vi "Modelo planta H2_V2.vi"() -> ()   [LabVIEW 2024]
uses:
  <vilib>/Modbus/master/Create Master Instance (TCP).vi
  <vilib>/Modbus/master/Modbus Master.lvclass
  <vilib>/OPCUA/NI OPC UA Client.lvlib
  SALICRU_MODBUS.lvlib
  S7-1200_OPCUA.lvlib
panel:
  out "x-y 2":u32
  out "error out 2":errorcluster
  out "error out":errorcluster
  in  "stop":bool
  out "x-y":u32
  in  "Tab Control":enum32{"Vista General", "Producción", "Energía"}(tab)
  out "EV5":bool caption="Not initialized"
  out "EV6":bool caption="Not initialized"
  out "EV4":bool caption="Not initialized"
  out "EV2":bool caption="Not initialized"
  out "EV3":bool caption="Idle"
  out "EV1":bool caption="Stand By"
  out "E2.2":bool caption="Not initialized"
  out "E2.3":bool caption="Not initialized"
  out "E2.14 2":bool caption="Not initialized"
  out "E1.2":bool caption="Not initialized"
  out "E1.3":bool caption="Idle"
  out "E1.1":bool caption="Stand By"
  out "Prod electrolizadores (display) 2":dbl format="%#.4g"
  out "Potenica Solar (Display) 2":dbl format="%#.2f"
  out "masa total G g 2":dbl format="%#.0f"
  out "P alta 2":dbl format="%.2f"
  out "P baja 2":dbl format="%.2f"
  out "masa total P g  2":dbl format="%#.1f"
  in  "SAI":bool caption="Line"
  out "Potenica Solar (Display) 3":dbl format="%#.2f"
  out "E2.1":bool caption="Not initialized"
  out "E2.2":bool caption="Not initialized"
  out "E1.2 2":bool caption="Idle"
  out "E1.1,2":bool caption="Stand By"
  out "E2.1 3":bool caption="Not initialized"
  out "E1.2":bool caption="Not initialized"
  out "Producció d'hidrogen":dbl(graph)
  out "Energia solar no utilitzada":dbl(graph)
  out "Pressió tanc baixa":dbl(graph)
  out "Potenica Solar (Display)":dbl format="%#.2f"
  out "Producción FC":dbl format="%#_2g"
  out "Prod electrolizadores (display)":dbl format="%#.4g"
  out "P baja":dbl format="%.2f"
  out "masa total G g":dbl format="%#.0f"
  out "Potència inversor solar":dbl(graph)
  out "Watimetro ARPA":dbl format="%#.1f"
  out "masa total P g":dbl format="%#.1f"
  out "Compresor":bool
  out "P alta":dbl format="%.2f"
  out "Tèrmic\nExtractors":bool
  out "Relé Seguretat":bool
  out "Sobretensions":bool
  out "Baliza verde":bool
  out "Baliza amarilla":bool
  out "Baliza roja":bool
  out "H2 generado Total":dbl format="%#.1f"
  out "Producción Solar toral":dbl format="%#.1f"
  out "Energía acum H2 verde":dbl format="%#.1f"
  out "H2 consumido en el lab":dbl=182.6 format="%#.1f"
  out "Energía solar diaría":dbl format="%#.1f"
  out "H2 generado dia":dbl format="%#.1f"
  out "Tank":dbl(slide) scale=0.0..10.0
  out "P tanq alta (barg)":dbl(graph)
  in  "Energía acum H2 verde inicio":dbl=527.0
  in  "Producción Solar total inicio":dbl=3421.0
  in  "H2 generado inicio":dbl=202.8
  out "g H2 consumidos por la FC":dbl
  out "g comprimidos":dbl
  in  "Caudal compresor":dbl
  out "P tanq baja (barg)":dbl(graph)
  in  "Presión ini Tanq baba":dbl=28.0
  in  "Presión ini Tanq alta":dbl=220.0
  out "Energía Solar no usada (kWh)":dbl(graph)
  out "H2 acumulado diario (g)":dbl(graph)
  out "Producción instalan (g/s)":dbl(graph)
  out "Electroli ON":dbl(graph)
  out "Potencia Consumo electroli instan. (kW)":dbl(graph)
  out "Producción diaria (g)":dbl
  out "Producción instalan (g/s)":dbl
  out "Electroli ON":dbl
  out "Potencia Solar Instanta (kW)":dbl(graph)
  # "g"
  # "bar"
  # "bar"
  # "kg"
  # "kWh"
  # "kWh"
  # "ESTADO ELECTROVÁLVULAS"
  # "SAI PLANTA"
  # "EV1:"
  # "EV4:"
  # "Modo:"
  # "EV2:"
  # "EV5:"
  # "EV3:"
  # "EV6:"
  # "ESTADO ELECTROLIZADORES"
  # "E1.1:"
  # "E2,1:"
  # "E1.2:"
  # "E2,2:"
  # "E2,3:"
  # "E1.3:"
  # "Electrolizadores"
  # "Producción\nElectrolizadores:"
  # "g/s"
  # "Inversor solar:"
  # "Energía solar:"
  # "kW"
  # "Tanque Alta"
  # "Presión:"
  # "barg"
  # "g"
  # "Capacidad:"
  # "Tanque Baja"
  # "Presión:"
  # "barg"
  # "g"
  # "Capacidad:"
  # "SAI:"
  # "Potencia (%):"
  # "%"
  # "Seguretat"
  # "H2 baixa pressió"
  # "H2 alta pressió"
  # "barg"
  # "Tanc baixa pressió"
  # "Tanc alta pressió"
  # "Compressor"
  # "barg"
  # "Solar"
  # "Fuel Cell"
  # "kW"
  # "kW"
  # "g"
  # "g"
  # "Electrolizadores"
  # "g/s"
  # "Xarxa electrica"
  # "-"
  # "+"
  # "kW de xarxa"
  # "Producció total d'hidrogen"
  # "Producció d'hidrogen diària"
  # "g"
  # "kg"
  # "Producció total d'energia solar"
  # "Energia solar produïda diària"
  # "kWh"
  # "kWh"
  # "Energia acumulada per H2 verd"
  # "Consum de H2 Lab diari"
  # "g"
  # "kWh"
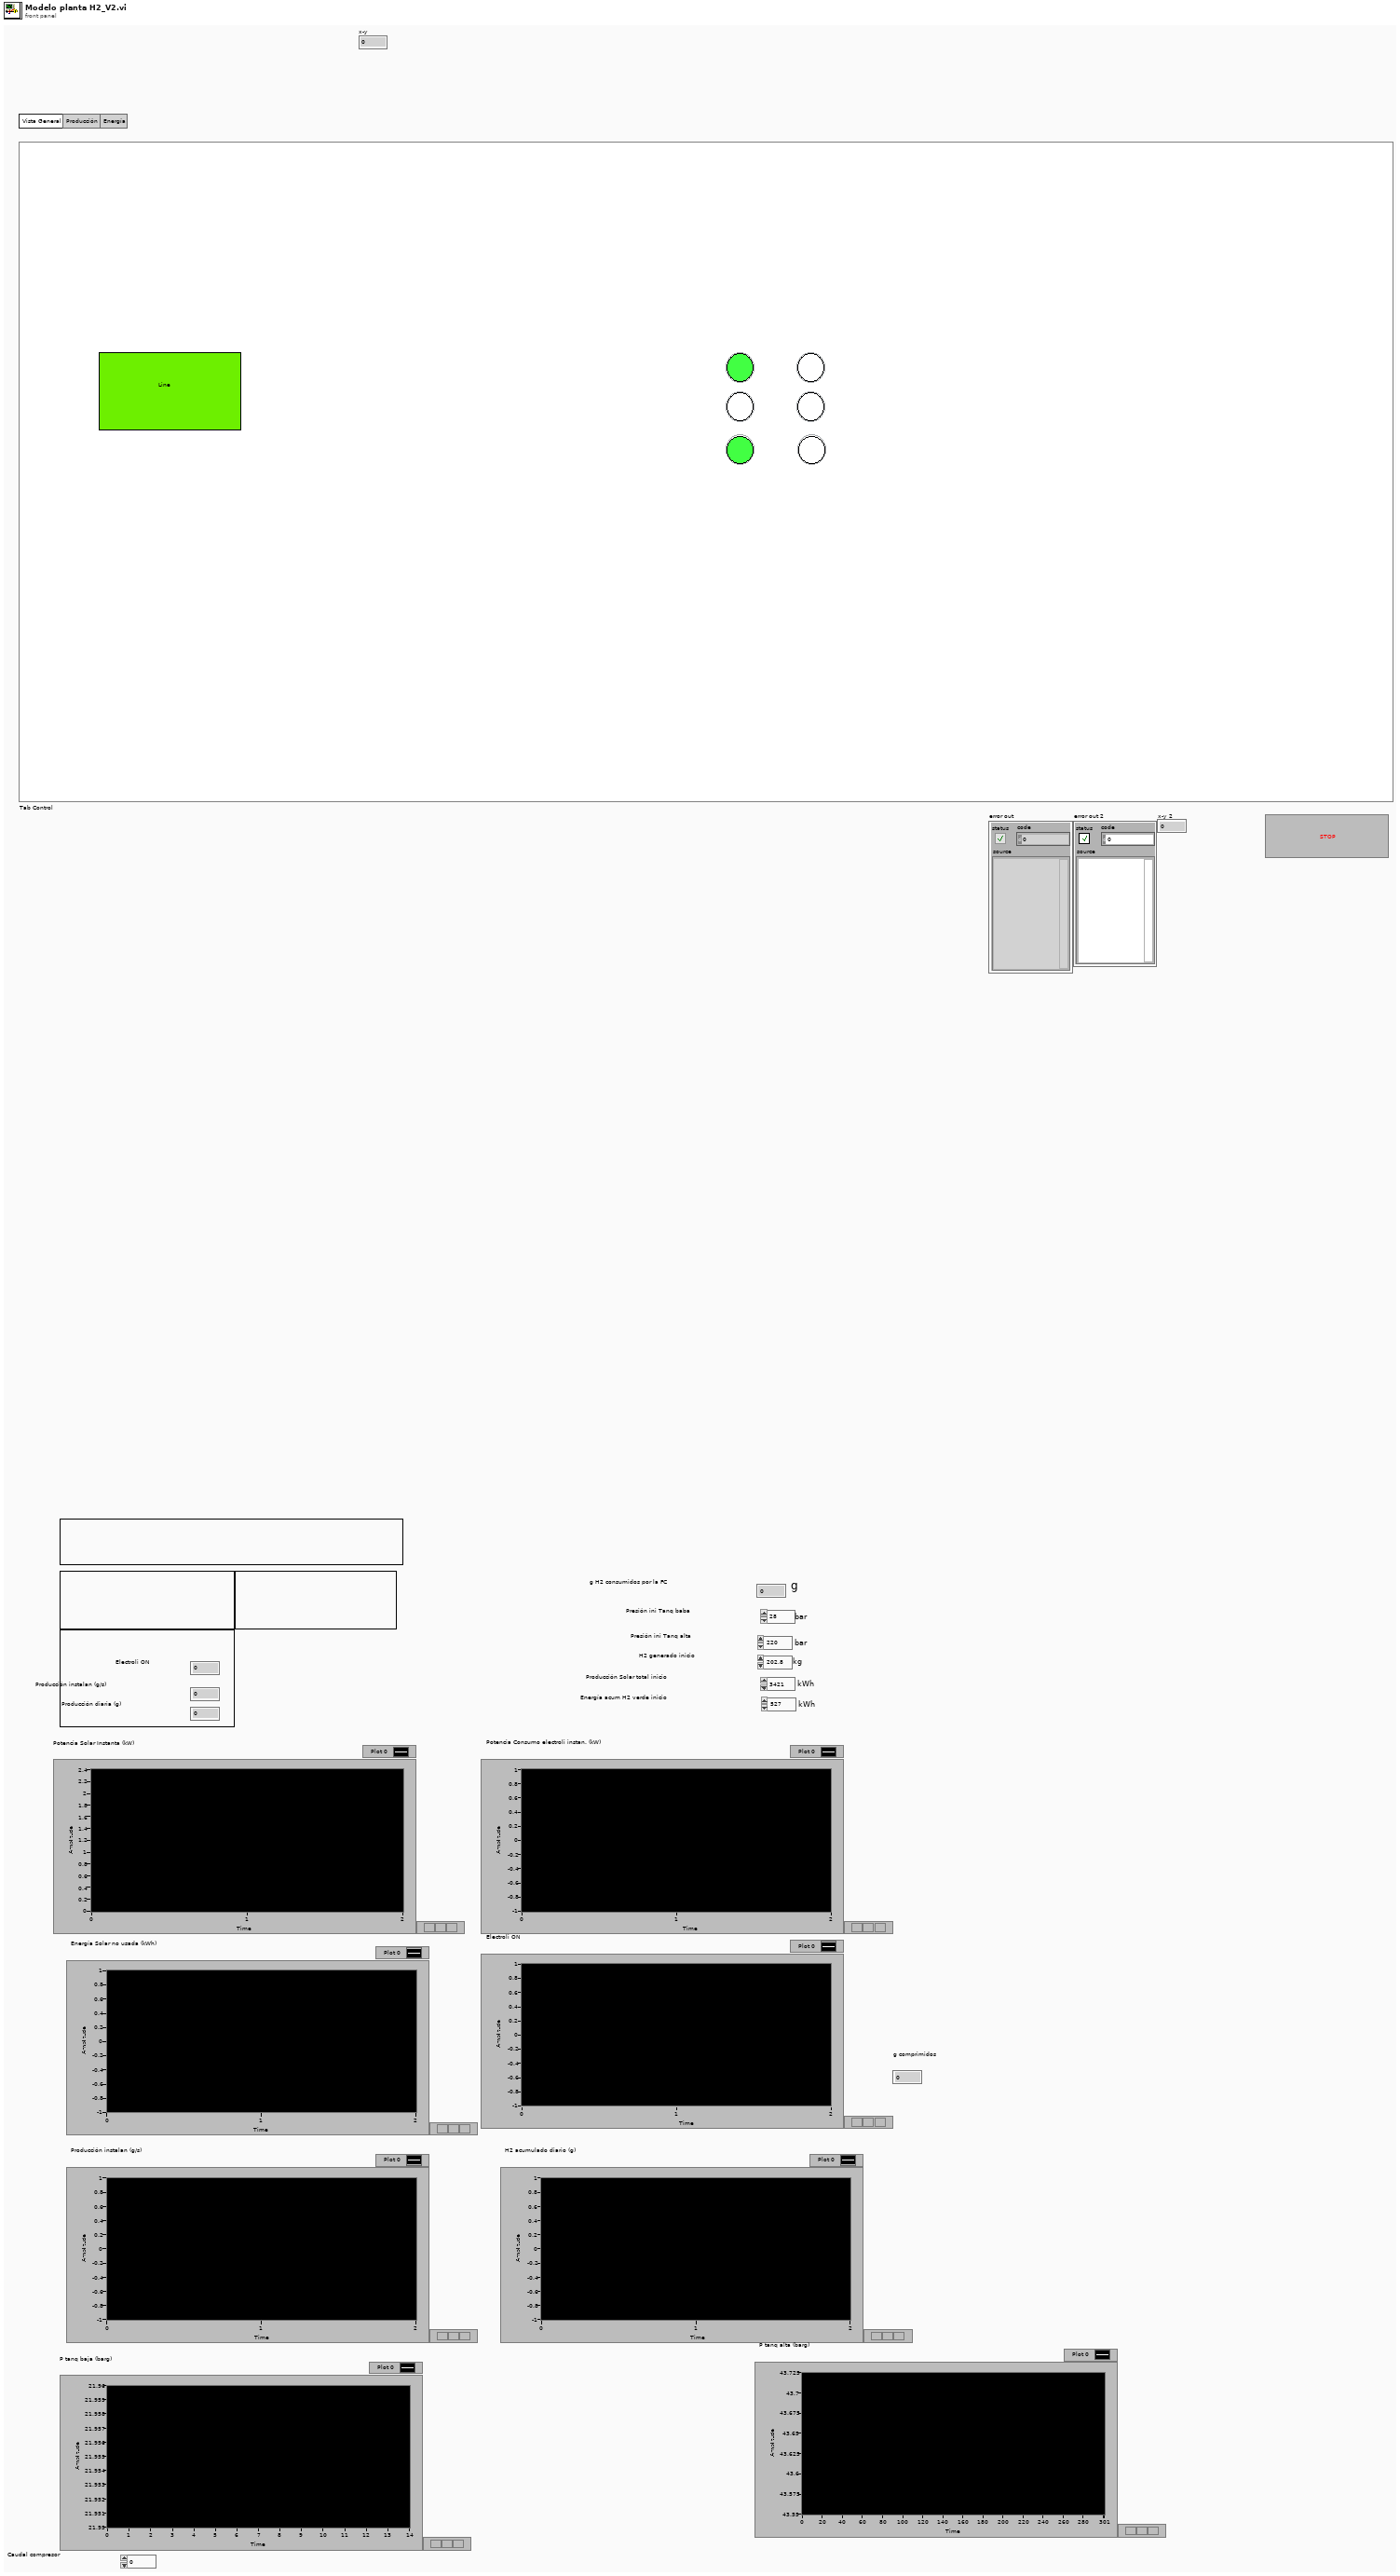
[diagram p1: front panel]
types:
  T1 = cluster{"message mode":enum16{"None", "Sign", "Sign and Encrypt"}, "security":enum16{"Basic256", "Basic128Rsa15"}}
  T2 = typedef "OPC UA Client Refnum.ctl" = refnum<k21>
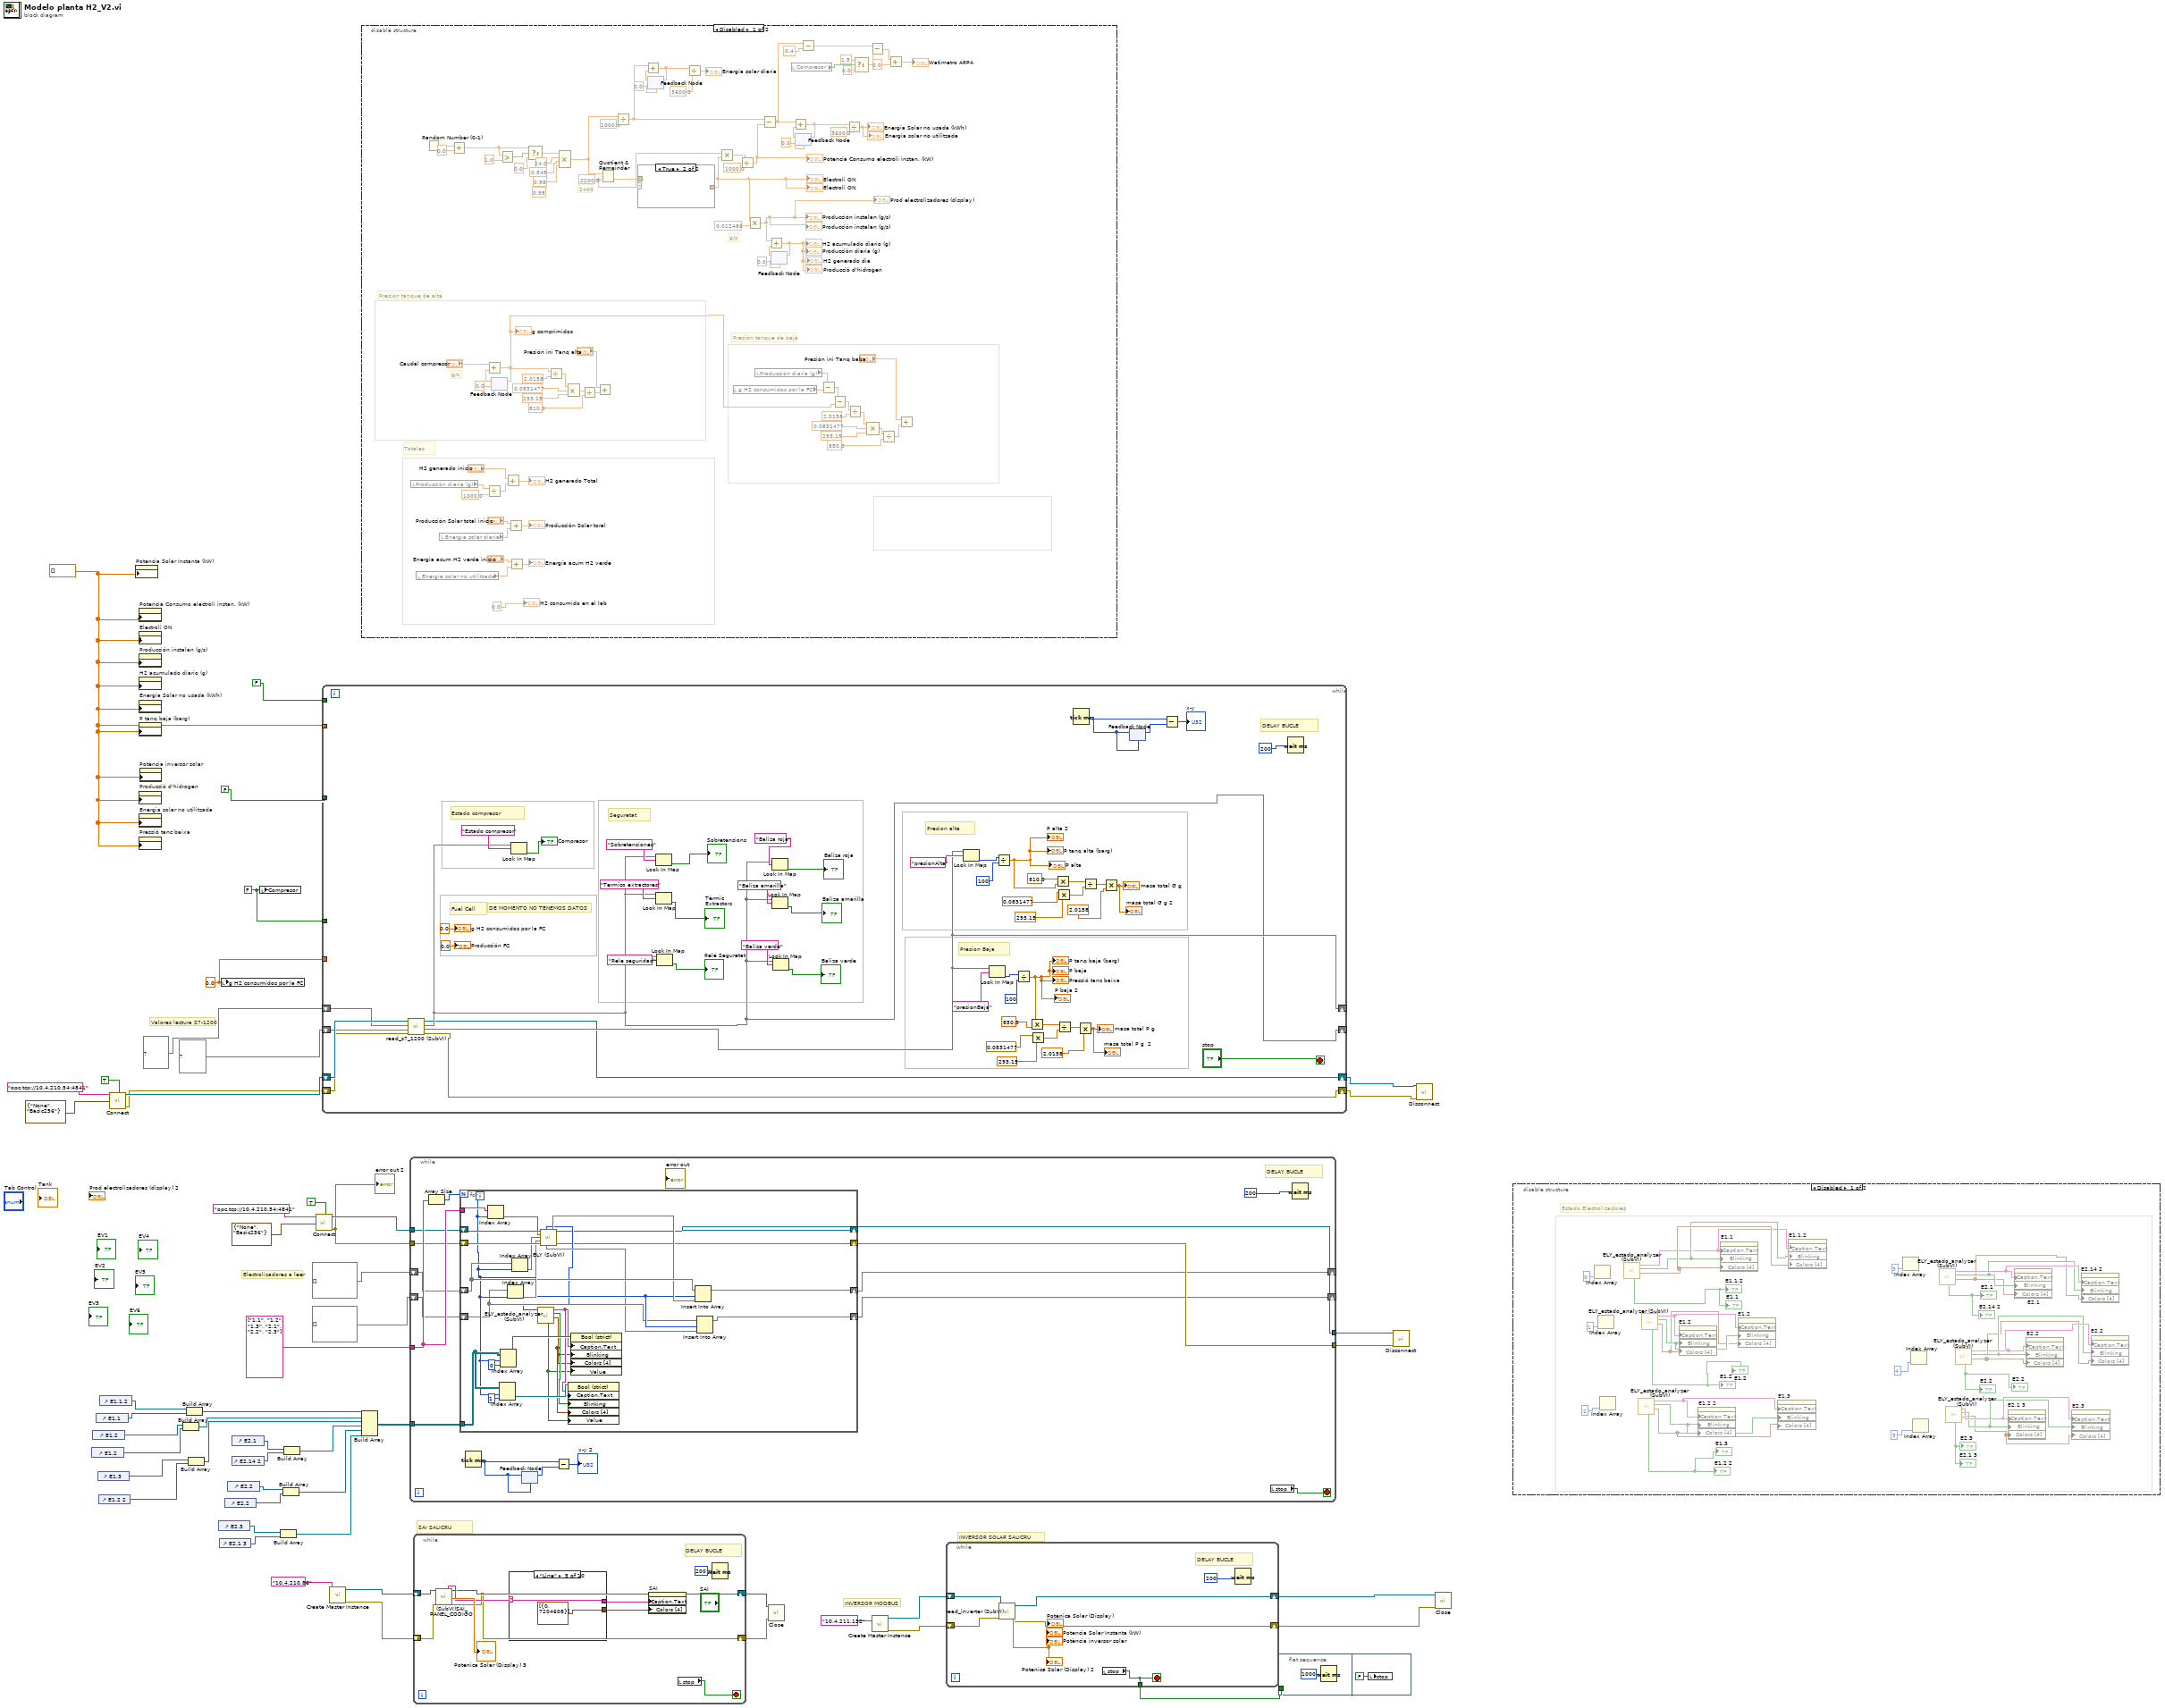
[diagram p0: block diagram]
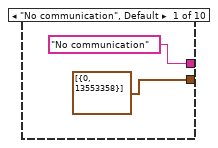
[diagram p5: hidden frame]
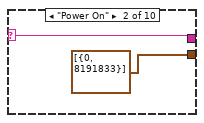
[diagram p6: hidden frame]
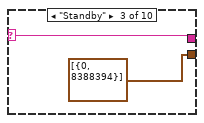
[diagram p7: hidden frame]
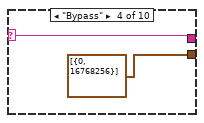
[diagram p8: hidden frame]
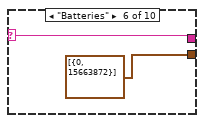
[diagram p9: hidden frame]
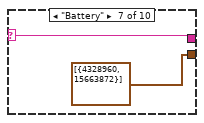
[diagram p10: hidden frame]
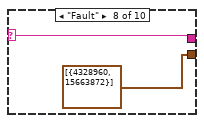
[diagram p11: hidden frame]
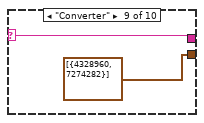
[diagram p12: hidden frame]
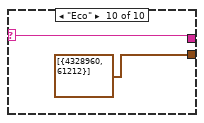
[diagram p13: hidden frame]
diagram:
  w50 = 0.0 ("g H2 consumidos por la FC")
  w51 = FALSE ("Compresor")
  w53 = dbl[] [] ("History Data")
  # "Valores lectura S7-1200"
  # "Electrolizadores a leer"
  # "INVERSOR SOLAR SALICRU"
  # "SAI SALICRU"
  # "INVERSOR MODBUS"
  n1 = control-ref of="E1.2"() -> (w21:refnum<vi>)
  n2 = control-ref of="E1.2"() -> (w20:refnum<vi>)
  n3 = control-ref of="E1.1"() -> (w18:refnum<vi>)
  n4 = control-ref of="E1.3"() -> (w16:refnum<vi>)
  n5 = control-ref of="E1.2 2"() -> (w15:refnum<vi>)
  n6 = control-ref of="E1.1,2"() -> (w17:refnum<vi>)
  n7 = call <vilib>:"Connect.vi"("trust any server (F)"=TRUE, "security policy"=T1 {"message mode"=enum."None", "security"=enum."Basic256"}, "server endpoint URL"="opc.tcp://10.4.210.54:4841") -> ("error out"=w31:errorcluster, "OPC UA client refnum out"=w32:T2)  [unwired: 6 in, 1 out]
  n8 = property on="Potencia Solar Instanta (kW)" class="WFChart (strict)"("History Data"=w53) -> ()  [unwired: 2 in, 2 out]
  n9 = property on="Potencia Consumo electroli instan. (kW)" class="WFChart (strict)"("History Data"=w53) -> ()  [unwired: 2 in, 2 out]
  n10 = property on="Electroli ON" class="WFChart (strict)"("History Data"=w53) -> ()  [unwired: 2 in, 2 out]
  n11 = property on="Producción instalan (g/s)" class="WFChart (strict)"("History Data"=w53) -> ()  [unwired: 2 in, 2 out]
  n12 = property on="H2 acumulado diario (g)" class="WFChart (strict)"("History Data"=w53) -> ()  [unwired: 2 in, 2 out]
  n13 = property on="Energía Solar no usada (kWh)" class="WFChart (strict)"("History Data"=w53) -> ()  [unwired: 2 in, 2 out]
  n14 = property on="P tanq baja (barg)" class="WFChart (strict)"("History Data"=w53) -> ()  [unwired: 2 in, 2 out]
  n15 = property on="Producció d'hidrogen" class="WFChart (strict)"("History Data"=w53) -> ()  [unwired: 2 in, 2 out]
  n16 = property on="Energia solar no utilitzada" class="WFChart (strict)"("History Data"=w53) -> ()  [unwired: 2 in, 2 out]
  n17 = property on="Pressió tanc baixa" class="WFChart (strict)"("History Data"=w53) -> ()  [unwired: 2 in, 2 out]
  n18 = property on="Potència inversor solar" class="WFChart (strict)"("History Data"=w53) -> ()  [unwired: 2 in, 2 out]
  n19 = Build Array(w20, w21) -> (w22:refnum<vi>[])
  n20 = Build Array(w17, w18) -> (w19:refnum<vi>[])
  n21 = Build Array(w16, w15) -> (w14:refnum<vi>[])
  n22 = control-ref of="E2.3"() -> (w7:refnum<vi>)
  n23 = control-ref of="E2.1 3"() -> (w6:refnum<vi>)
  n24 = local write "g H2 consumidos por la FC"(w50) -> ()
  n25 = control-ref of="E2.2"() -> (w9:refnum<vi>)
  n26 = control-ref of="E2.2"() -> (w10:refnum<vi>)
  n27 = control-ref of="E2.1"() -> (w13:refnum<vi>)
  n28 = control-ref of="E2.14 2"() -> (w12:refnum<vi>)
  n29 = local write "Compresor"(w51) -> ()
  n30 = Build Array(w7, w6) -> (w5:refnum<vi>[])
  n31 = Build Array(w10, w9) -> (w8:refnum<vi>[])
  n32 = Build Array(w13, w12) -> (w11:refnum<vi>[])
  n33 = call <vilib>:"Connect.vi"("trust any server (F)"=TRUE, "security policy"=T1 {"message mode"=enum."None", "security"=enum."Basic256"}, "server endpoint URL"="opc.tcp://10.4.210.54:4841") -> ("error out"=w26:errorcluster, "OPC UA client refnum out"=w27:T2)  [unwired: 6 in, 1 out]
  "error out 2" <- w26
  n34 = while {
    tunnel: w53 -> [_]
    tunnel: FALSE ("Manual") -> [_]
    tunnel: w51 -> [_]
    tunnel: FALSE ("stop 2") -> [_]
    tunnel: w50 -> [_]
    shift-right: [w56] -> w25
    shift-left: w32 -> [w107]
    shift-right: [w55] -> w24
    shift-left: w31 -> [w106]
    shift-right: [w58] -> _
    shift-left: map{string, bool} {} ("Coils in") -> [w60]
    shift-right: [w59] -> _
    shift-left: map{string, i32} {} ("Values in") -> [w61]
    stop <- "stop" stop-if-true
    # "DELAY BUCLE"
    # "Seguretat"
    # "Presion Baja"
    # "Presion alta"
    # "DE MOMENTO NO TENEMOS DATOS"
    # "Fuel Cell"
    # "Estado compresor"
    n35 = call "read_s7_1200 (SubVI).vi"("error in (no error)"=w106, "Coils in"=w60, "Values in"=w61, "Refnum in"=w107) -> ("error out"=w55:errorcluster, "VALUES READ"=w59:map{string, i32}, "Coils read"=w58:map{string, bool}, "Refnum out"=w56:T2)  [unwired: 4 in]
    n36 = Look In Map(map=w58, key="Estado compresor") -> (value=→"Compresor":bool)  [unwired: 1 in, 1 out]
    n37 = Look In Map(map=w58, key="Sobretensiones") -> (value=→"Sobretensions":bool)  [unwired: 1 in, 1 out]
    n38 = Look In Map(map=w58, key="Termico extractores") -> (value=→"Tèrmic\nExtractors":bool)  [unwired: 1 in, 1 out]
    n39 = Look In Map(map=w58, key="Rele seguridad") -> (value=→"Relé Seguretat":bool)  [unwired: 1 in, 1 out]
    n40 = Look In Map(map=w58, key="Baliza roja") -> (value=→"Baliza roja":bool)  [unwired: 1 in, 1 out]
    n41 = Look In Map(map=w58, key="Baliza amarilla") -> (value=→"Baliza amarilla":bool)  [unwired: 1 in, 1 out]
    n42 = Look In Map(map=w58, key="Baliza verde") -> (value=→"Baliza verde":bool)  [unwired: 1 in, 1 out]
    n43 = Look In Map(map=w59, key="presionAlta") -> (value=w87:i32)  [unwired: 1 in, 1 out]
    n44 = Look In Map(map=w59, key="presionBaja") -> (value=w85:i32)  [unwired: 1 in, 1 out]
    n45 = Divide(x=w87, y=100) -> (x/y=w68:dbl)
    "P tanq alta (barg)" <- w68
    "P alta" <- w68
    "P alta 2" <- w68
    n46 = Divide(x=w85, y=100) -> (x/y=w69:dbl)
    "P tanq baja (barg)" <- w69
    "P baja" <- w69
    "Pressió tanc baixa" <- w69
    "P baja 2" <- w69
    n47 = Multiply(x=w69, y=850.0) -> (x*y=w76:dbl)
    n48 = Multiply(x=0.0831477 ("y"), y=293.15) -> (x*y=w74:dbl)
    n49 = Multiply(x=810.0 ("y"), y=w68) -> (x*y=w79:dbl)
    n50 = Multiply(x=0.0831477 ("y"), y=293.15) -> (x*y=w82:dbl)
    n51 = Divide(x=w76, y=w74) -> (x/y=w73:dbl)
    n52 = Tick Count (ms)() -> (millisecond timer value=w65:u32)
    n53 = Multiply(x=w73, y=2.0158) -> (x*y=→"masa total P g" →"masa total P g  2":dbl)
    n54 = Divide(x=w79, y=w82) -> (x/y=w83:dbl)
    n55 = Multiply(x=w83, y=2.0158) -> (x*y=→"masa total G g" →"masa total G g 2":dbl)
    n56 = feedback-in #1(w65) -> ()
    n57 = feedback #1(w65) -> (w64:u32)
    n58 = Subtract(x=w65, y=w64) -> (x-y=→"x-y":u32)
    n59 = Wait (ms)(milliseconds to wait=u32 200) -> ()  [unwired: 1 out]
    "Producción FC" <- 0.0 ("Producción FC")
    "g H2 consumidos por la FC" <- 0.0 ("g H2 consumidos por la FC")
  }
  n60 = call-poly <vilib>:"Create Master Instance.vi"("address"="10.4.210.86") -> ("error out"=w43:errorcluster, "TCP master instance"=w44:refnum<class "Modbus Master.lvclass">)  [unwired: 9 in]
  n61 = disable-structure shown="Disabled" {
    frame Disabled {
      (unwired) 0.95 ("f")
      w124 = 2200.0 ("y")
      # "Totales"
      # "g/s"
      # "2400"
      # "g/s"
      # "Presión tanque de alta"
      # "Presión tanque de baja"
      n62 = local read "Producción diaria (g)"() -> (w119:dbl)
      n63 = local read "Energia solar no utilitzada"() -> (w110:dbl)
      n64 = Random Number (0-1)() -> (number: 0 to 1=w135:dbl)
      n65 = local read "Energía solar diaría"() -> (w114:dbl)
      n66 = Add(x=w135, y=0.0) -> (x+y=w136:dbl)
      n67 = Divide(x=w119, y=1000.0) -> (x/y=w118:dbl)
      n68 = feedback #2(0.0) -> (w182:dbl)
      n69 = Add(x="Caudal compresor", y=w182) -> (x+y=w178:dbl)
      "g comprimidos" <- w178
      n70 = feedback-in #2(w178) -> ()
      n71 = Greater?(x=w136, y=1.0) -> (0:w137:bool)
      n72 = Add(x="H2 generado inicio", y=w118) -> (x+y=→"H2 generado Total":dbl)
      n73 = Add(x="Producción Solar total inicio", y=w114) -> (x+y=→"Producción Solar toral":dbl)
      n74 = Add(x="Energía acum H2 verde inicio", y=w110) -> (x+y=→"Energía acum H2 verde":dbl)
      n75 = Select(t=w136, s=w137, f=0.0) -> (s? t:f=w138:dbl)
      n76 = Divide(x=w178, y=2.0158) -> (x/y=w176:dbl)
      n77 = Compound Arithmetic op=MULTIPLY(w138, 24.0 ("f"), 0.545 ("f"), 0.98 ("f")) -> (w146:dbl)
      n78 = Compound Arithmetic op=MULTIPLY(w176, 0.0831477 ("y"), 293.15 ("y")) -> (w186:dbl)
      n79 = Divide(x=w186, y=810.0) -> (x/y=w185:dbl)
      n80 = Add(x="Presión ini Tanq alta", y=w185) -> (x+y=w180:dbl)
      n81 = Quotient & Remainder(x=w146, y=w124) -> (floor(x/y)=w145:dbl)  [unwired: 1 out]
      n82 = Divide(x=w146, y=1000.0) -> (x/y=w161:dbl)
      n83 = case shown="True" {
        selector: _ -> [_ _]
        tunnel: w145 -> [w190 _]
        tunnel: [w190 _] -> w151
        frame False {
        }
        frame True {
        }
      }
      "Electroli ON" <- w151
      "Electroli ON" <- w151
      n84 = feedback #3(0.0) -> (w160:dbl)
      n85 = Add(x=w161, y=w160) -> (x+y=w159:dbl)
      n86 = feedback-in #3(w159) -> ()
      n87 = Divide(x=w159, y=3600.0) -> (x/y=→"Energía solar diaría":dbl)
      n88 = Multiply(x=w124, y=w151) -> (x*y=w147:dbl)
      n89 = local read "g H2 consumidos por la FC"() -> (w165:dbl)
      n90 = Divide(x=w147, y=1000.0) -> (x/y=w148:dbl)
      "Potencia Consumo electroli instan. (kW)" <- w148
      n91 = Multiply(x=w151, y=0.012486) -> (x*y=w149:dbl)
      "Producción instalan (g/s)" <- w149
      "Producción instalan (g/s)" <- w149
      "Prod electrolizadores (display)" <- w149
      n92 = local read "Producción diaria (g)"() -> (w167:dbl)
      n93 = Subtract(x=w161, y=w148) -> (x-y=w152:dbl)
      n94 = feedback #4(0.0) -> (w142:dbl)
      n95 = Add(x=w149, y=w142) -> (x+y=w163:dbl)
      "Producción diaria (g)" <- w163
      "H2 acumulado diario (g)" <- w163
      "Producció d'hidrogen" <- w163
      "H2 generado dia" <- w163
      n96 = feedback-in #4(w163) -> ()
      n97 = local read "Compresor"() -> (w153:bool)
      n98 = feedback #5(0.0) -> (w143:dbl)
      n99 = Add(x=w152, y=w143) -> (x+y=w144:dbl)
      n100 = feedback-in #5(w144) -> ()
      n101 = Subtract(x=w152, y=0.4) -> (x-y=w155:dbl)
      n102 = Subtract(x=w167, y=w165) -> (x-y=w166:dbl)
      n103 = Subtract(x=w166, y=w178) -> (x-y=w170:dbl)
      n104 = Divide(x=w144, y=3600.0) -> (x/y=→"Energía Solar no usada (kWh)" →"Energia solar no utilitzada":dbl)
      n105 = Divide(x=w170, y=2.0158) -> (x/y=w175:dbl)
      n106 = Select(t=1.5, s=w153, f=0.0 ("t")) -> (s? t:f=w154:dbl)
      n107 = Compound Arithmetic op=MULTIPLY(w175, 0.0831477 ("y"), 293.15 ("y")) -> (w173:dbl)
      n108 = Subtract(x=w155, y=w154) -> (x-y=w156:dbl)
      n109 = Divide(x=w173, y=850.0) -> (x/y=w169:dbl)
      n110 = Add(x=w156, y=0.0) -> (x+y=→"Watimetro ARPA":dbl)
      n111 = Add(x="Presión ini Tanq baba", y=w169) -> (x+y=w164:dbl)
      "H2 consumido en el lab" <- 0.0 ("H2 consumido en el lab")
    }
    frame Enabled {
    }
  }
  n112 = Build Array(w19, w22, w14, w11, w8, w5) -> (w4:refnum<vi>[][])
  n113 = while {
    tunnel: string[] ["1.1", "1.2", "1.3", "2.1", "2.2", "2.3"] -> [w204]
    tunnel: w27 -> [w203]
    tunnel: w26 -> [w202]
    tunnel: [w201] -> w23
    tunnel: w4 -> [w197]
    tunnel: [w195] -> w3
    shift-right: [w192] -> _
    shift-left: map{string, dbl}[] [] -> [w194]
    shift-right: [w191] -> _
    shift-left: map{string, dbl}[] [] -> [w193]
    stop <- w206 stop-if-true
    # "DELAY BUCLE"
    n114 = Array Size(array=w204) -> (size(s)=w205:i32)
    n115 = for {
      N: w205 -> [_]
      shift-right: [w208] -> w201
      shift-left: w203 -> [w221]
      shift-right: [w207] -> w195
      shift-left: w202 -> [w220]
      tunnel: w204 -> [w231]
      tunnel: w197 -> [w230]
      shift-right: [w214] -> w192
      shift-left: w194 -> [w216]
      shift-right: [w210] -> w191
      shift-left: w193 -> [w212]
      i -> [w213]
      n116 = Index Array(array=w231, index=w213) -> (element=w219:string)
      n117 = Index Array(array=w230, index (row)=w213, index (col)=1 ("disabled index (col)")) -> (element=w226:refnum<vi>)
      n118 = Index Array(array=w230, index (row)=w213, index (col)=0 ("disabled index (col)")) -> (element=w227:refnum<vi>)
      n119 = Index Array(array=w212, index=w213) -> (element=w217:map{string, dbl})
      n120 = Index Array(array=w216, index=w213) -> (element=w218:map{string, dbl})
      n121 = call "ELY (SubVI).vi"("Refnum in"=w221, "Electrolizador"=w219, "Produccion in"=w218, "Medidas in"=w217, "error in (no error)"=w220) -> ("Estado"=w209:u16, "Produccion"=w215:map{string, dbl}, "Refnum out"=w208:T2, "Medidas"=w211:map{string, dbl}, "error out"=w207:errorcluster)  [unwired: 3 in, 3 out]
      n122 = call "ELY_estado_analyzer (SubVI).vi"("Numeric"=w209) -> ("Colors [4]"=w223:cluster{u32, u32}[], "Boolean 2"=w224:bool, "Caption.Text"=w225:string, "Boolean"=w222:bool)  [unwired: 7 in]
      n123 = property class="Bool (strict)"(reference=w226, "Caption.Text"=w225, "Blinking"=w224, "Colors [4]"=w223, "Value"=w222) -> ()  [unwired: 1 in, 2 out]
      n124 = property class="Bool (strict)"(reference=w227, "Caption.Text"=w225, "Blinking"=w224, "Colors [4]"=w223, "Value"=w222) -> ()  [unwired: 1 in, 2 out]
      n125 = Insert Into Array(array=w216, index=w213, new element=w215) -> (w214:map{string, dbl}[])
      n126 = Insert Into Array(array=w212, index=w213, new element=w211) -> (w210:map{string, dbl}[])
    }
    n127 = Tick Count (ms)() -> (millisecond timer value=w200:u32)
    n128 = feedback #6(w200) -> (w199:u32)
    n129 = feedback-in #6(w200) -> ()
    n130 = Subtract(x=w200, y=w199) -> (x-y=→"x-y 2":u32)
    n131 = local read "stop"() -> (w206:bool)
    n132 = Wait (ms)(milliseconds to wait=u32 200) -> ()  [unwired: 1 out]
  }
  n133 = while {
    shift-right: [w235] -> w42
    shift-left: w44 -> [w237]
    shift-right: [w234] -> w41
    shift-left: w43 -> [w236]
    stop <- w233 stop-if-true
    # "DELAY BUCLE"
    n134 = call "(SubVI)SAI_PANEL_CODIGO.vi"("Modbus Master in"=w237, "error in (no error)"=w236) -> ("Work mode"=w238:string, "Modbus Master out"=w235:refnum<class "Modbus Master.lvclass">, "Porcentaje P"=→"Potenica Solar (Display) 3":dbl, "error out"=w234:errorcluster)  [unwired: 4 in, 10 out]
    n135 = case shown="\"Line\"" w238 {
      selector: w238 -> [_ w245 w247 w249 w251 w253 w255 w257 w259 w261]
      tunnel: ["No communication" w245 w247 w249 w251 w253 w255 w257 w259 w261] -> w239
      tunnel: [cluster{u32, u32}[] [{0, 13553358}] ("Colors [4]") cluster{u32, u32}[] [{0, 8191833}] ("Colors [4]") cluster{u32, u32}[] [{0, 8388394}] ("Colors [4]") cluster{u32, u32}[] [{0, 16768256}] ("Colors [4]") cluster{u32, u32}[] [{0, 7204608}] ("Colors [4]") cluster{u32, u32}[] [{0, 15663872}] ("Colors [4]") cluster{u32, u32}[] [{4328960, 15663872}] ("Colors [4]") cluster{u32, u32}[] [{4328960, 15663872}] ("Colors [4]") cluster{u32, u32}[] [{4328960, 7274282}] ("Colors [4]") cluster{u32, u32}[] [{4328960, 61212}] ("Colors [4]")] -> w240
      frame "No communication", Default {
      }
      frame "Power On" {
      }
      frame "Standby" {
      }
      frame "Bypass" {
      }
      frame "Line" {
      }
      frame "Batteries" {
      }
      frame "Battery" {
      }
      frame "Fault" {
      }
      frame "Converter" {
      }
      frame "Eco" {
      }
    }
    n136 = property on="SAI" class="Bool"("Caption.Text"=w239, "Colors [4]"=w240) -> ()  [unwired: 2 in, 2 out]
    n137 = local read "stop"() -> (w233:bool)
    n138 = Wait (ms)(milliseconds to wait=u32 200) -> ()  [unwired: 1 out]
  }
  n139 = call-dynamic "Close.vi"("error in (no error)"=w41, "Modbus master in"=w42) -> ()  [unwired: 9 in, 1 out]
  n140 = call-poly <vilib>:"Create Master Instance.vi"("address"="10.4.211.152") -> ("error out"=w38:errorcluster, "TCP master instance"=w39:refnum<class "Modbus Master.lvclass">)  [unwired: 9 in]
  n141 = while {
    shift-right: [w264] -> w37
    shift-left: w39 -> [w266]
    shift-right: [w267] -> w40
    shift-left: w38 -> [w265]
    tunnel: [w263] -> w36
    stop <- w263 stop-if-true
    # "DELAY BUCLE"
    n142 = call "read_inverter (SubVI).vi"("error in (no error)"=w265, "Modbus Master in"=w266) -> ("error out"=w267:errorcluster, "Inverter kW"=→"Potencia Solar Instanta (kW)" →"Potenica Solar (Display)" →"Potència inversor solar" →"Potenica Solar (Display) 2":dbl, "Modbus Master out"=w264:refnum<class "Modbus Master.lvclass">)  [unwired: 7 in]
    n143 = local read "stop"() -> (w263:bool)
    n144 = Wait (ms)(milliseconds to wait=u32 200) -> ()  [unwired: 1 out]
  }
  n145 = flat-sequence {
    tunnel: w36 -> [_]
    frame #0 {
      n146 = Wait (ms)(milliseconds to wait=u32 1000) -> ()  [unwired: 1 out]
    }
    frame #1 {
      n147 = local write "stop"(FALSE ("stop")) -> ()
    }
  }
  n148 = call <vilib>:"Disconnect.vi"("error in (no error)"=w3, "OPC UA client refnum in"=w23) -> ()  [unwired: 9 in, 1 out]
  n149 = call <vilib>:"Disconnect.vi"("error in (no error)"=w24, "OPC UA client refnum in"=w25) -> ()  [unwired: 9 in, 1 out]
  n150 = call-dynamic "Close.vi"("error in (no error)"=w40, "Modbus master in"=w37) -> ()  [unwired: 9 in, 1 out]
  n151 = disable-structure shown="Disabled" {
    frame Disabled {
      # "Estado Electrolizadores"
      n152 = Index Array(index=0) -> ()  [unwired: 1 in, 1 out]
      n153 = Index Array(index=1) -> ()  [unwired: 1 in, 1 out]
      n154 = Index Array(index=2) -> ()  [unwired: 1 in, 1 out]
      n155 = call "ELY_estado_analyzer (SubVI).vi"() -> ("Colors [4]"=w300:cluster{u32, u32}[], "Boolean 2"=w299:bool, "Caption.Text"=w298:string, "Boolean"=→"E1.1" →"E1.1,2":bool)  [unwired: 8 in]
      n156 = call "ELY_estado_analyzer (SubVI).vi"() -> ("Colors [4]"=w289:cluster{u32, u32}[], "Boolean 2"=w290:bool, "Caption.Text"=w291:string, "Boolean"=→"E1.2 2" →"E1.3":bool)  [unwired: 8 in]
      n157 = call "ELY_estado_analyzer (SubVI).vi"() -> ("Colors [4]"=w293:cluster{u32, u32}[], "Boolean 2"=w294:bool, "Caption.Text"=w295:string, "Boolean"=→"E1.2" →"E1.2":bool)  [unwired: 8 in]
      n158 = property on="E1.2" class="Bool (strict)"("Caption.Text"=w295, "Blinking"=w294, "Colors [4]"=w293) -> ()  [unwired: 2 in, 2 out]
      n159 = property on="E1.2 2" class="Bool (strict)"("Caption.Text"=w291, "Blinking"=w290, "Colors [4]"=w289) -> ()  [unwired: 2 in, 2 out]
      n160 = property on="E1.1" class="Bool (strict)"("Caption.Text"=w298, "Blinking"=w299, "Colors [4]"=w300) -> ()  [unwired: 2 in, 2 out]
      n161 = property on="E1.2" class="Bool (strict)"("Caption.Text"=w295, "Blinking"=w294, "Colors [4]"=w293) -> ()  [unwired: 2 in, 2 out]
      n162 = property on="E1.3" class="Bool (strict)"("Caption.Text"=w291, "Blinking"=w290, "Colors [4]"=w289) -> ()  [unwired: 2 in, 2 out]
      n163 = property on="E1.1,2" class="Bool (strict)"("Caption.Text"=w298, "Blinking"=w299, "Colors [4]"=w300) -> ()  [unwired: 2 in, 2 out]
      n164 = Index Array(index=3) -> ()  [unwired: 1 in, 1 out]
      n165 = Index Array(index=4) -> ()  [unwired: 1 in, 1 out]
      n166 = Index Array(index=5) -> ()  [unwired: 1 in, 1 out]
      n167 = call "ELY_estado_analyzer (SubVI).vi"() -> ("Colors [4]"=w285:cluster{u32, u32}[], "Boolean 2"=w286:bool, "Caption.Text"=w287:string, "Boolean"=→"E2.1" →"E2.14 2":bool)  [unwired: 8 in]
      n168 = call "ELY_estado_analyzer (SubVI).vi"() -> ("Colors [4]"=w277:cluster{u32, u32}[], "Boolean 2"=w278:bool, "Caption.Text"=w279:string, "Boolean"=→"E2.3" →"E2.1 3":bool)  [unwired: 8 in]
      n169 = call "ELY_estado_analyzer (SubVI).vi"() -> ("Colors [4]"=w281:cluster{u32, u32}[], "Boolean 2"=w282:bool, "Caption.Text"=w283:string, "Boolean"=→"E2.2" →"E2.2":bool)  [unwired: 8 in]
      n170 = property on="E2.1 3" class="Bool (strict)"("Caption.Text"=w279, "Blinking"=w278, "Colors [4]"=w277) -> ()  [unwired: 2 in, 2 out]
      n171 = property on="E2.1" class="Bool (strict)"("Caption.Text"=w287, "Blinking"=w286, "Colors [4]"=w285) -> ()  [unwired: 2 in, 2 out]
      n172 = property on="E2.2" class="Bool (strict)"("Caption.Text"=w283, "Blinking"=w282, "Colors [4]"=w281) -> ()  [unwired: 2 in, 2 out]
      n173 = property on="E2.3" class="Bool (strict)"("Caption.Text"=w279, "Blinking"=w278, "Colors [4]"=w277) -> ()  [unwired: 2 in, 2 out]
      n174 = property on="E2.14 2" class="Bool (strict)"("Caption.Text"=w287, "Blinking"=w286, "Colors [4]"=w285) -> ()  [unwired: 2 in, 2 out]
      n175 = property on="E2.2" class="Bool (strict)"("Caption.Text"=w283, "Blinking"=w282, "Colors [4]"=w281) -> ()  [unwired: 2 in, 2 out]
    }
    frame Enabled {
    }
  }
